vi "IR Opo Main.vi"() -> ()   [LabVIEW 2016]
uses:
  <vilib>/vision/NI_Vision_Development_Module.lvlib
  D:/Fabrizio/Labview Projects/VersionControlled/Laser Ablation Capture Software/uc480DotNet.dll
  Laser Ablation Capture Software/uc480DotNet.dll
  System.Windows.Forms
  <vilib>/Utility/miscctls.llb/LVBoundsTypeDef.ctl
  <vilib>/Utility/config.llb/NI_LVConfig.lvlib
  <vilib>/regexp/Match Regular Expression.xnode
panel:
  in  "Load ROI":bool
  in  "Save current ROI":bool
  in  "Call Last ROI":bool
  in  "Circle?":bool=TRUE
  out "Axis 2 group":i32
  out "Axis 1 group":i32
  in  "Microscope/Capture \nstatus button":bool=TRUE
  in  "X travel":dbl min=0.0 max=50.0 step=0.0001
  in  "Y travel":dbl min=0.0 max=150.0 step=0.0001
  in  "Laser Status":bool
  in  "SINGLE SHOT":bool
  in  "Repetition\nRate (Hz)":dbl=2.34 min=1.0 max=20.0 step=0.01 format="%.2g"
  out "Laser Com Delay":i32
  out "VISA Laser port":string
  in  "Acceleration \n(mm/s²)":dbl=20.0
  out "Camera Status":string="Load parameter"
  in  "Save configuration":bool
  in  "Stages status":bool
  in  "Transparency":u8 max=80 step=1
  in  "Overlay MSI Image":bool
  in  "Home Axes":bool
  out "Axis 2 Offset":dbl
  out "Axis 1 Offset":dbl
  out "Acceleration":dbl
  out "Velocity":dbl
  in  "Axis Initial Parameters":T1={"Velocity (units/seconds)"=1.0, "Acceleration (units/seconds²)"=20.0, "Minimum Jerk Time (seconds)"=0.005, "Maximum Jerk Time (seconds)"=0.009} {"Maximum Jerk Time (seconds)" format="%.6e"; "Minimum Jerk Time (seconds)" format="%.6e"; "Acceleration (units/seconds²)" format="%.6e"; "Velocity (units/seconds)" format="%.6e"}
  out "Axis 2":string
  out "Axis 1":string
  out "XPS_Address":string
  in  "Axes Manual Control":bool
  out "ROI Area \n(mm2)":dbl=4.035870075999999
  out "Laser on/off array":bool[][](array[boolean])
  out "Commands array":string[][](array[string])
  in  "Exit Camera":bool
  in  "Width (px)":i32=240
  in  "Y offset":i32=406 step=1
  in  "X offset":i32=693 step=1
  out "Processi time (sec)":i32=117
  in  "Processing time unit":string(combo)="sec"
  out "Process time":dbl=117.0
  in  "Mode":i32(ring) items=["RGB 32"=0, "RGB 24"=1, "Y8 Monochrom"=6]
  in  "Camera":refnum<k24>(container)
  in  "Init Camera":bool
  in  "Start Live":bool
  in  "Stop Live":bool
  in  "Load Parameter":bool
  out "Error Out":errorcluster caption="error"
  out "Bits/Pixel":i32=32
  out "Width":i32=1280
  out "Height":i32=1024
  out "Serial Number":string="4102944807"
  in  "Camera ID":i32
  in  "Zoom":dbl(ring)=1.5 items=["4X"=4.0, "2X"=2.0, "1.5X"=1.5, "1.25X"=1.25, "1X"=1.0]
  in  "Gain Boost":bool=TRUE
  in  "Snapshot":bool
  out "Output":picture
  in  "Exposure":dbl(slide)=99.80425000000001 min=0.06241666666666667 max=99.80425000000001 step=0.06241666666666667 scale=0.06241666666666667..99.80425000000001 scale format="%#.3g"
  in  "Framerate":dbl(slide)=10.002522802986672 min=0.47411700449083627 max=15.001275108384213 step=0.014032998230481021 scale=0.47411700449083627..15.001275108384213 scale format="%#.3g"
  in  "Pixelclock":i32(slide)=24 min=5 max=40 step=1 scale=5.0..40.0
  in  "error in (no error)":errorcluster
  out "error out":errorcluster
  in  "Precision (%)":dbl=1.0 min=1.0 max=100.0 step=1.0 format="%#_3g"
  in  "Process Image":bool
  in  "Pixel size":dbl=12.19 step=0.01
  in  "Speed (µm/s)":i32=1000
  in  "Heigth (px)":i32=240
  in  "Height  step \ndivider":i32=2
  out "ROI container\nheigth (µm)":i32=2267
  out "ROI container\nwidth (µm)":i32=2267
  out "Source":T2(plugin-control)
  in  "Open \nManual":bool
  in  "Capture":bool
  out "Log":string
  out "Laser Operation":bool
  in  "LASER":bool
  in  "LAMP":bool
  in  "EXIT":bool
  # "Laser Control"
  # "Stages Control"
  # "Camera Control"
  # "ROI Processing"
  # "Laser spot size and position"
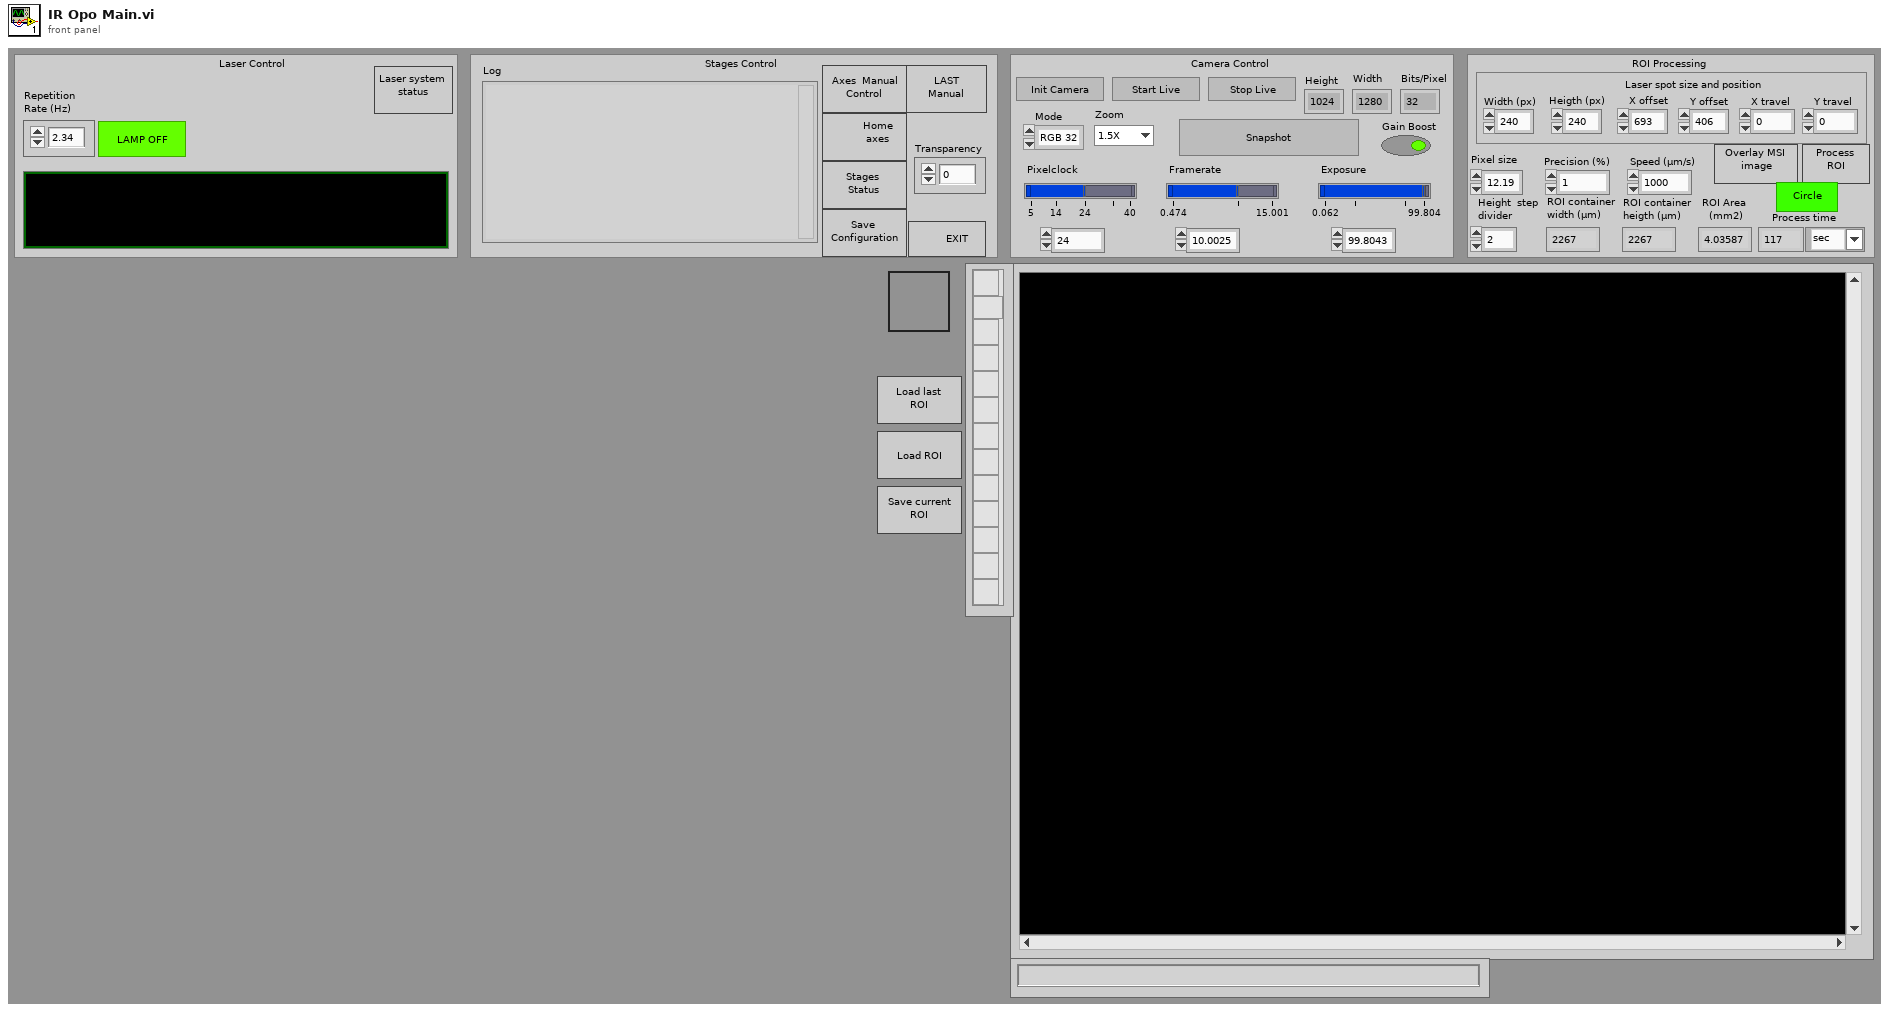
[diagram p1: front panel]
types:
  T1 = cluster{"Velocity (units/seconds)":dbl, "Acceleration (units/seconds²)":dbl, "Minimum Jerk Time (seconds)":dbl, "Maximum Jerk Time (seconds)":dbl}
  T2 = typedef "IMAQ Image.ctl" = refnum<image>
  T3 = typedef "LVBoundsTypeDef.ctl" = cluster{"Width":u32, "Height":u32}
  T4 = enum8{"Enabled", "Disabled", "Disabled and Grayed Out"}
  T5 = typedef "NI_LVConfig.lvlib/Config Data RefNum.ctl" = refnum<k1>
  T6 = enum16{"open", "replace", "create", "open or create", "replace or create", "replace or create with confirmation"}
  T7 = enum32{"Invalid", "Standard", "Closed", "Hidden", "Minimized", "Maximized"}
  T8 = enum32{"invalid app kind", "Development System", "Run Time System", "Student Edition", "Embedded LabVIEW", "Evaluation", "Custom"}
  T9 = cluster{"connection TCP":refnum<k5>, "LogTo File":bool, "Log File refnum":refnum<file>, "no error if error log":bool}
  T10 = typedef "Image Type" = u32
  T11 = cluster{"Global Rectangle":i32[], "Contours":cluster{"Contour Type":u32, "ROI Type":u32, "Points":i32[]}[]}
  T12 = cluster{"Global Rectangle[0]":i32, "Global Rectangle[1]":i32}
  T13 = typedef "ROI Descriptor" = cluster{"Global Rectangle":i32[], "Contours":cluster{"ID":enum32{"External", "Internal"}, "Type":u32, "Coordinates":i32[]}[]}
  T14 = cluster{"ID":enum32{"External", "Internal"}, "Type":u32, "Coordinates":i32[]}[]
  T15 = cluster{"ID":enum32{"External", "Internal"}, "Type":u32, "Coordinates":i32[]}
  T16 = cluster{"Contour Type":u32, "ROI Type":u32, "Points":i32[]}[]
  T17 = cluster{"Contour Type":u32, "ROI Type":u32, "Points":i32[]}
diagram:
  w35 = 1 items=["None", "FixedSingle", "Fixed3D"] ("BorderStyle")
  # "Button and controls"
  # "Camera control buttons"
  n1 = property class="PictureBox"(reference="Camera", "BorderStyle"=w35, "Width"=853, "Height"=682) -> (reference out=w23:refnum<k24>, error out=w24:errorcluster)  [unwired: 1 in]
  n2 = property class="PictureBox"(reference=w23, error in=w24) -> (reference out=w22:refnum<k24>, error out=w21:errorcluster, "Handle"=w20:refnum<k24>)
  n3 = while "Camera Control" {
    shift-right: [w52] -> _
    shift-left: w21 -> [w58]
    shift-right: [w55] -> _
    shift-left: _ -> [w48]
    shift-right: [w50] -> _
    shift-left: w22 -> [w51]
    tunnel: w20 -> [w49]
    stop <- w56 stop-if-true
    # ".NetReference"
    # ".Net Reference"
    n4 = event shown="[1] Timeout" {
      selector: _ -> [_ _]
      dyn-events: _ -> [_ _]
      timeout: 0 -> [_ _]
      event "Load Parameter", "Start Live": Mouse Down {
        n5 = event-data() -> ()  [unwired: 1 in, 2 out]
      }
      event Timeout {
        n6 = event-data() -> ()  [unwired: 1 in, 2 out]
      }
    }
    n7 = event shown="[1] Timeout" {
      selector: _ -> [_ _]
      dyn-events: _ -> [_ _]
      timeout: 0 -> [_ _]
      tunnel: [w72 w83] -> w59
      tunnel: w58 -> [w82 w83]
      tunnel: w48 -> [w81 _]
      event "Pixelclock": Value Change; "Pixelclock": Mouse Move; "Pixelclock": Key Down; "Pixelclock": Mouse Up {
        n8 = event-data() -> ("CtlRef"=w74:refnum<vi>)  [unwired: 1 in, 3 out]
        n9 = call "uc480_SubVI_Example_GetFramerate.vi"(".NET (Reference)"=w81, "Error In"=w82) -> ("Framerate"=w80:dbl, "Inc"=w79:dbl, "Min"=w77:dbl, "Max"=w78:dbl, "error out"=w76:errorcluster)  [unwired: 9 in]
        n10 = property on="Framerate" class="Slide (strict)"(error in=w76, "Value"=w80, "Increment"=w79, "Minimum"=w77, "Maximum"=w78) -> (error out=w75:errorcluster)  [unwired: 1 in, 1 out]
        n11 = property on="Framerate" class="Slide (strict)"(error in=w75, "Scale.Increment"=w79, "Scale.Minimum"=w77, "Scale.Maximum"=w78) -> (error out=w73:errorcluster)  [unwired: 1 in, 1 out]
        n12 = Close Reference(reference=w74, error in (no error)=w73) -> (error out=w72:errorcluster)
      }
      event Timeout {
        n13 = event-data() -> ()  [unwired: 1 in, 2 out]
      }
    }
    n14 = case shown="False" "Load Parameter" {
      tunnel: ["" "Load parameter"] -> w65
      frame False {
      }
      frame True {
      }
    }
    n15 = case shown="False" "Init Camera" {
      tunnel: ["" "Init camera"] -> w69
      frame False {
      }
      frame True {
      }
    }
    n16 = case shown="False" "Exit Camera" {
      tunnel: ["" "Exit camera"] -> w63
      frame False {
      }
      frame True {
      }
    }
    n17 = event shown="[1] Timeout" {
      selector: _ -> [_ _]
      dyn-events: _ -> [_ _]
      timeout: 0 -> [_ _]
      tunnel: w59 -> [w94 w95]
      tunnel: [w84 w95] -> w61
      tunnel: w48 -> [w93 _]
      event "Pixelclock", "Framerate": Value Change; "Pixelclock", "Framerate": Mouse Move; "Pixelclock", "Framerate": Key Down; "Pixelclock", "Framerate": Mouse Up {
        n18 = event-data() -> ("CtlRef"=w86:refnum<vi>)  [unwired: 1 in, 3 out]
        n19 = call "uc480_SubVI_Example_GetExposure.vi"(".NET (Reference)"=w93, "Error In"=w94) -> ("Exposure"=w90:dbl, "Inc"=w89:dbl, "Min"=w88:dbl, "Max"=w87:dbl, "Error out"=w91:errorcluster)  [unwired: 9 in]
        n20 = property on="Exposure" class="Slide (strict)"(error in=w91, "Value"=w90, "Increment"=w89, "Minimum"=w88, "Maximum"=w87) -> (error out=w92:errorcluster)  [unwired: 1 in, 1 out]
        n21 = property on="Exposure" class="Slide (strict)"(error in=w92, "Scale.Increment"=w89, "Scale.Minimum"=w88, "Scale.Maximum"=w87) -> (error out=w85:errorcluster)  [unwired: 1 in, 1 out]
        n22 = Close Reference(reference=w86, error in (no error)=w85) -> (error out=w84:errorcluster)
      }
      event Timeout {
        n23 = event-data() -> ()  [unwired: 1 in, 2 out]
      }
    }
    n24 = case shown="False" "Start Live" {
      tunnel: ["" "Start live"] -> w68
      frame False {
      }
      frame True {
      }
    }
    n25 = case shown="False" "Stop Live" {
      tunnel: ["" "Stop live"] -> w64
      frame False {
      }
      frame True {
      }
    }
    n26 = local read "Camera Status"() -> (w45:string)
    n27 = Concatenate Strings(w69, w68, w65, w64, w63) -> (→"Camera Status":string)
    n28 = case shown="Default" w45 {
      tunnel: w48 -> [w138 w178 w236 w278 w458 w517]
      tunnel: w61 -> [w141 w179 w237 w288 w457 w518]
      tunnel: [w112 w177 w245 w287 w416 w516] -> w55
      tunnel: [w113 w176 w246 w286 w453 w514] -> w54
      tunnel: [FALSE FALSE TRUE FALSE FALSE FALSE] -> w56
      tunnel: w51 -> [w111 w170 w218 w270 w411 w507]
      tunnel: [w111 w170 w217 w269 w411 w507] -> w50
      tunnel: w49 -> [_ _ _ w266 _ _]
      frame "Load parameter" {
        # "SubVI Example for \nMemory allocation"
        # "Is acquisition running?"
        # "Load Parameter"
        n29 = property class="Camera"(reference=w138, error in=w141) -> (error out=w146:errorcluster, "Acquisition"=w145:refnum<k24>)  [unwired: 1 out]
        n30 = invoke class="Acquisition" method="HasStarted"(reference=w145, error in=w146) -> (reference out=w142:refnum<k24>, error out=w144:errorcluster, "bValue"=w140:bool)  [unwired: 2 in, 1 out]
        n31 = control-ref of="Start Live"() -> (w136:refnum<vi>)
        n32 = invoke class="Acquisition" method="ToString"(reference=w142, error in=w144) -> (reference out=w108:refnum<k24>, error out=w107:errorcluster, "ToString"=w143:string)  [unwired: 1 in]
        n33 = property class="Bool"(reference=w136, "Disabled"=u8 0 ("Deaktiviert")) -> (reference out=w110:refnum<vi>, error out=w109:errorcluster)  [unwired: 1 in]
        n34 = Close Reference(reference=w108, error in (no error)=w107) -> (error out=w106:errorcluster)
        n35 = Close Reference(reference=w110, error in (no error)=w109) -> ()  [unwired: 1 out]
        n36 = call "uc480_Error_Handling.vi"("Error String"=w143, "Error In"=w106) -> ("Error Out"=w139:errorcluster)  [unwired: 9 in]
        n37 = case shown="False" w140 {
          tunnel: w139 -> [w154 w161]
          tunnel: w138 -> [w152 w162]
          tunnel: [w153 w161] -> w137
          tunnel: [w152 w162] -> w112
          frame False {
            n38 = property class="Camera"(reference=w152, error in=w154) -> (error out=w156:errorcluster, "Parameter"=w155:refnum<k24>)  [unwired: 1 out]
            n39 = invoke class="Parameter" method="Load"(reference=w155, error in=w156, "strFilename"="") -> (reference out=w158:refnum<k24>, error out=w159:errorcluster, "Load"=w151:i32)  [unwired: 1 in, 1 out]
            n40 = invoke class="Parameter" method="ToString"(reference=w158, error in=w159) -> (reference out=w148:refnum<k24>, error out=w150:errorcluster, "ToString"=w160:string)  [unwired: 1 in]
            n41 = Close Reference(reference=w148, error in (no error)=w150) -> (error out=w149:errorcluster)
            n42 = call "uc480_Error_Handling.vi"("Error Code"=w151, "Error String"=w160, "Error In"=w149) -> ("Error Out"=w153:errorcluster)  [unwired: 8 in]
          }
          frame True {
          }
        }
        n43 = call "uc480_SubVI_Example_MemoryAllocation.vi"(".NET (Reference)"=w112, "Error In"=w137) -> ("Error Out"=w114:errorcluster)  [unwired: 13 in, 4 out]
        n44 = call "uc480_SubVI_Example_GetPixelClock.vi"(".NET (Reference)"=w112, "Error In"=w114) -> ("Pixel Clock"=w115:i32, "Inc"=w117:i32, "Min"=w118:i32, "Max"=w119:i32, "error out"=w116:errorcluster)  [unwired: 9 in]
        n45 = property on="Pixelclock" class="Slide (strict)"(error in=w116, "Value"=w115, "Increment"=w117, "Minimum"=w118, "Maximum"=w119) -> (error out=w120:errorcluster)  [unwired: 1 in, 1 out]
        n46 = property on="Pixelclock" class="Slide (strict)"(error in=w120, "Scale.Increment"=w117, "Scale.Minimum"=w118, "Scale.Maximum"=w119) -> (error out=w121:errorcluster)  [unwired: 1 in, 1 out]
        n47 = call "uc480_SubVI_Example_GetFramerate.vi"(".NET (Reference)"=w112, "Error In"=w121) -> ("Framerate"=w124:dbl, "Inc"=w125:dbl, "Min"=w126:dbl, "Max"=w127:dbl, "error out"=w123:errorcluster)  [unwired: 9 in]
        n48 = property on="Framerate" class="Slide (strict)"(error in=w123, "Value"=w124, "Increment"=w125, "Minimum"=w126, "Maximum"=w127) -> (error out=w122:errorcluster)  [unwired: 1 in, 1 out]
        n49 = property on="Framerate" class="Slide (strict)"(error in=w122, "Scale.Increment"=w125, "Scale.Minimum"=w126, "Scale.Maximum"=w127) -> (error out=w128:errorcluster)  [unwired: 1 in, 1 out]
        n50 = call "uc480_SubVI_Example_GetExposure.vi"(".NET (Reference)"=w112, "Error In"=w128) -> ("Exposure"=w131:dbl, "Inc"=w132:dbl, "Min"=w133:dbl, "Max"=w134:dbl, "Error out"=w129:errorcluster)  [unwired: 9 in]
        n51 = property on="Exposure" class="Slide (strict)"(error in=w129, "Value"=w131, "Increment"=w132, "Minimum"=w133, "Maximum"=w134) -> (error out=w130:errorcluster)  [unwired: 1 in, 1 out]
        n52 = property on="Exposure" class="Slide (strict)"(error in=w130, "Scale.Increment"=w132, "Scale.Minimum"=w133, "Scale.Maximum"=w134) -> (error out=w113:errorcluster)  [unwired: 1 in, 1 out]
      }
      frame "Stop live" {
        # "Is acquisition running?"
        # "Stop Acquisition"
        n53 = property class="Camera"(reference=w178, error in=w179) -> (error out=w186:errorcluster, "Acquisition"=w185:refnum<k24>)  [unwired: 1 out]
        n54 = invoke class="Acquisition" method="HasStarted"(reference=w185, error in=w186) -> (reference out=w180:refnum<k24>, error out=w182:errorcluster, "bValue"=w184:bool)  [unwired: 2 in, 1 out]
        n55 = control-ref of="Load Parameter"() -> (w174:refnum<vi>)
        n56 = control-ref of="Start Live"() -> (w171:refnum<vi>)
        n57 = invoke class="Acquisition" method="ToString"(reference=w180, error in=w182) -> (reference out=w163:refnum<k24>, error out=w165:errorcluster, "ToString"=w181:string)  [unwired: 1 in]
        n58 = property class="Bool"(reference=w174, "Disabled"=u8 0 ("Deaktiviert")) -> (reference out=w169:refnum<vi>, error out=w168:errorcluster)  [unwired: 1 in]
        n59 = property class="Bool"(reference=w171, "Disabled"=u8 0 ("Deaktiviert")) -> (reference out=w167:refnum<vi>, error out=w166:errorcluster)  [unwired: 1 in]
        n60 = Close Reference(reference=w163, error in (no error)=w165) -> (error out=w164:errorcluster)
        n61 = Close Reference(reference=w169, error in (no error)=w168) -> ()  [unwired: 1 out]
        n62 = Close Reference(reference=w167, error in (no error)=w166) -> ()  [unwired: 1 out]
        n63 = call "uc480_Error_Handling.vi"("Error String"=w181, "Error In"=w164) -> ("Error Out"=w183:errorcluster)  [unwired: 9 in]
        n64 = case shown="True" w184 {
          tunnel: [w188 w207] -> w176
          tunnel: w183 -> [w188 w208]
          tunnel: w178 -> [w187 w200]
          tunnel: [w187 w200] -> w177
          frame False {
          }
          frame True {
            n65 = property class="Camera"(reference=w200, error in=w208) -> (error out=w204:errorcluster, "Acquisition"=w205:refnum<k24>)  [unwired: 1 out]
            n66 = invoke class="Acquisition" method="Stop"(reference=w205, error in=w204) -> (reference out=w202:refnum<k24>, error out=w203:errorcluster, "Stop"=w201:i32)  [unwired: 1 in]
            n67 = invoke class="Acquisition" method="ToString"(reference=w202, error in=w203) -> (reference out=w197:refnum<k24>, error out=w199:errorcluster, "ToString"=w206:string)  [unwired: 1 in]
            n68 = Close Reference(reference=w197, error in (no error)=w199) -> (error out=w198:errorcluster)
            n69 = call "uc480_Error_Handling.vi"("Error Code"=w201, "Error String"=w206, "Error In"=w198) -> ("Error Out"=w207:errorcluster)  [unwired: 8 in]
            n70 = Get Date/Time In Seconds() -> (seconds since 1Jan1904=w195:timestamp)
            n71 = Format Date/Time String(time format string (%c)="%m/%d/%y - %I:%M %p  ", seconds (now)=w195) -> (date/time string=w196:string)  [unwired: 1 in]
            n72 = Concatenate Strings(w196, "Camera stopped", "\r") -> (w191:string)
            n73 = invoke on="Log" class="Str" method="Append String"("string"=w191) -> (error out=w189:errorcluster)  [unwired: 3 in, 3 out]
            n74 = property on="Log" class="Str"(error in=w189, "Text.Scroll Position"=u32 500000) -> ()  [unwired: 1 in, 2 out]
          }
        }
      }
      frame "Exit camera" {
        # "Close .Net Reference"
        # "Is acquisition running?"
        # "Stop Acquisition"
        # "Close Camera"
        n75 = property class="Camera"(reference=w236, error in=w237) -> (error out=w244:errorcluster, "Acquisition"=w243:refnum<k24>)  [unwired: 1 out]
        n76 = invoke class="Acquisition" method="HasStarted"(reference=w243, error in=w244) -> (reference out=w238:refnum<k24>, error out=w240:errorcluster, "bValue"=w242:bool)  [unwired: 2 in, 1 out]
        n77 = control-ref of="Load Parameter"() -> (w227:refnum<vi>)
        n78 = control-ref of="Init Camera"() -> (w229:refnum<vi>)
        n79 = control-ref of="Start Live"() -> (w228:refnum<vi>)
        n80 = control-ref of="Stop Live"() -> (w226:refnum<vi>)
        n81 = invoke class="Acquisition" method="ToString"(reference=w238, error in=w240) -> (reference out=w223:refnum<k24>, error out=w225:errorcluster, "ToString"=w239:string)  [unwired: 1 in]
        n82 = property class="Bool"(reference=w228, "Disabled"=u8 0 ("Deaktiviert")) -> (reference out=w212:refnum<vi>, error out=w211:errorcluster)  [unwired: 1 in]
        n83 = property class="Bool"(reference=w229, "Disabled"=u8 0 ("Deaktiviert")) -> (reference out=w210:refnum<vi>, error out=w209:errorcluster)  [unwired: 1 in]
        n84 = property class="Bool"(reference=w227, "Disabled"=u8 0 ("Deaktiviert")) -> (reference out=w214:refnum<vi>, error out=w213:errorcluster)  [unwired: 1 in]
        n85 = property class="Bool"(reference=w226, "Disabled"=u8 0 ("Deaktiviert")) -> (reference out=w216:refnum<vi>, error out=w215:errorcluster)  [unwired: 1 in]
        n86 = Close Reference ("Close Referenz")(reference=w223, error in (no error)=w225) -> (error out=w224:errorcluster)
        n87 = Close Reference(reference=w212, error in (no error)=w211) -> ()  [unwired: 1 out]
        n88 = Close Reference(reference=w210, error in (no error)=w209) -> ()  [unwired: 1 out]
        n89 = Close Reference(reference=w216, error in (no error)=w215) -> ()  [unwired: 1 out]
        n90 = Close Reference(reference=w214, error in (no error)=w213) -> ()  [unwired: 1 out]
        n91 = call "uc480_Error_Handling.vi"("Error String"=w239, "Error In"=w224) -> ("Error Out"=w241:errorcluster)  [unwired: 9 in]
        n92 = case shown="True" w242 {
          tunnel: [w253 w264] -> w234
          tunnel: w241 -> [w253 w265]
          tunnel: w236 -> [w252 w257]
          tunnel: [w252 w257] -> w235
          frame False {
          }
          frame True {
            n93 = property class="Camera"(reference=w257, error in=w265) -> (error out=w261:errorcluster, "Acquisition"=w262:refnum<k24>)  [unwired: 1 out]
            n94 = invoke class="Acquisition" method="Stop"(reference=w262, error in=w261) -> (reference out=w259:refnum<k24>, error out=w260:errorcluster, "Stop"=w258:i32)  [unwired: 1 in]
            n95 = invoke class="Acquisition" method="ToString"(reference=w259, error in=w260) -> (reference out=w254:refnum<k24>, error out=w256:errorcluster, "ToString"=w263:string)  [unwired: 1 in]
            n96 = Close Reference ("Close Referenz")(reference=w254, error in (no error)=w256) -> (error out=w255:errorcluster)
            n97 = call "uc480_Error_Handling.vi"("Error Code"=w258, "Error String"=w263, "Error In"=w255) -> ("Error Out"=w264:errorcluster)  [unwired: 8 in]
          }
        }
        n98 = invoke class="Camera" method="Exit"(reference=w235, error in=w234) -> (reference out=w245:refnum<k24>, error out=w248:errorcluster, "Exit"=w247:i32)  [unwired: 1 in]
        n99 = invoke class="Camera" method="ToString"(reference=w245, error in=w248) -> (error out=w249:errorcluster, "ToString"=w250:string)  [unwired: 1 in, 1 out]
        n100 = call "uc480_Error_Handling.vi"("Error Code"=w247, "Error String"=w250, "Error In"=w249) -> ("Error Out"=w222:errorcluster)  [unwired: 8 in]
        n101 = property class="PictureBox"(reference=w218, error in=w222, "Width"=853, "Height"=682) -> (reference out=w217:refnum<k24>, error out=w221:errorcluster)
        n102 = Close Reference ("Close Referenz")(reference=w245, error in (no error)=w221) -> (error out=w246:errorcluster)
      }
      frame Default {
        # "SubVI Example for Timing"
        # "Has acquisition started?"
        n103 = call "uc480_SubVI_Example_Timing.vi"(".NET (Reference)"=w278, "Pixelclock"="Pixelclock", "Exposure time"="Exposure", "Framerate"="Framerate", "Error In"=w288) -> ("Pixelclock"=w281:i32, "Exposure time"=w280:dbl, "Framerate"=w279:dbl, "Error Out"=w285:errorcluster)  [unwired: 7 in]
        n104 = property on="Framerate" class="Schieber (strikt)"(error in=w285, "Scale.RngStart"=w279) -> (error out=w284:errorcluster)  [unwired: 1 in, 1 out]
        n105 = property on="Exposure" class="Schieber (strikt)"(error in=w284, "Scale.RngStart"=w280) -> (error out=w283:errorcluster)  [unwired: 1 in, 1 out]
        n106 = property on="Pixelclock" class="Schieber (strikt)"(error in=w283, "Scale.RngStart"=w281) -> (error out=w282:errorcluster)  [unwired: 1 in, 1 out]
        n107 = property class="Camera"(reference=w278, error in=w282) -> (reference out=w271:refnum<k24>, error out=w294:errorcluster, "Acquisition"=w293:refnum<k24>)
        n108 = invoke class="Acquisition" method="HasStarted"(reference=w293, error in=w294) -> (reference out=w268:refnum<k24>, error out=w290:errorcluster, "HasStarted"=w289:i32, "bValue"=w267:bool)  [unwired: 2 in]
        n109 = invoke class="Acquisition" method="ToString"(reference=w268, error in=w290) -> (reference out=w272:refnum<k24>, error out=w292:errorcluster, "ToString"=w291:string)  [unwired: 1 in]
        n110 = call "uc480_Error_Handling.vi"("Error Code"=w289, "Error String"=w291, "Error In"=w292) -> ("Error Out"=w274:errorcluster)  [unwired: 8 in]
        n111 = Close Reference(reference=w272, error in (no error)=w274) -> (error out=w273:errorcluster)
        n112 = case "Show Image" shown="True" w267 {
          tunnel: [w298 w310] -> w286
          tunnel: w273 -> [w298 w338]
          tunnel: w271 -> [w297 w302]
          tunnel: [w297 w306] -> w287
          tunnel: w270 -> [w296 w327]
          tunnel: [w296 w304] -> w269
          tunnel: w266 -> [_ w334]
          frame False {
            (unwired) ""
          }
          frame True {
            n113 = local read "Height"() -> (w331:i32)
            n114 = local read "Width"() -> (w332:i32)
            n115 = Quotient & Remainder(x=w332, y="Zoom") -> (floor(x/y)=w329:dbl)  [unwired: 1 out]
            n116 = Quotient & Remainder(x=w331, y="Zoom") -> (floor(x/y)=w328:dbl)  [unwired: 1 out]
            n117 = To Long Integer(number=w329) -> (32bit integer=w301:i32)
            n118 = To Long Integer(number=w328) -> (32bit integer=w300:i32)
            n119 = property class="PictureBox"(reference=w327, error in=w338, "Width"=w301, "Height"=w300) -> (reference out=w304:refnum<k24>, error out=w333:errorcluster)
            n120 = property class="Camera"(reference=w302, error in=w333) -> (reference out=w303:refnum<k24>, error out=w340:errorcluster, "Memory"=w341:refnum<k24>)
            n121 = invoke class="Memory" method="GetActive"(reference=w341, error in=w340) -> (reference out=w335:refnum<k24>, error out=w336:errorcluster, "s32MemId"=w307:i32)  [unwired: 2 in, 1 out]
            n122 = property class="Camera"(reference=w303, error in=w336) -> (reference out=w315:refnum<k24>, error out=w339:errorcluster, "Display"=w324:refnum<k24>)
            n123 = invoke class="Display" method="Render"(reference=w324, error in=w339, "memID"=w307, "windowHandle"=w334) -> (reference out=w325:refnum<k24>, error out=w326:errorcluster)  [unwired: 1 in, 3 out]
            n124 = property class="Camera"(reference=w315, error in=w326) -> (reference out=w306:refnum<k24>, error out=w322:errorcluster, "Gain"=w320:refnum<k24>)
            n125 = property class="Gain"(reference=w320, error in=w322) -> (reference out=w321:refnum<k24>, error out=w317:errorcluster, "Hardware"=w316:refnum<k24>)
            n126 = property class="GainHardware"(reference=w316, error in=w317) -> (reference out=w313:refnum<k24>, error out=w318:errorcluster, "Boost"=w319:refnum<k24>)
            n127 = property class="GainBoost"(reference=w319, error in=w318, "Enabled"="Gain Boost") -> (reference out=w314:refnum<k24>, error out=w305:errorcluster)
            n128 = case "Snapshot control" shown="True" "Snapshot" {
              tunnel: w302 -> [_ w362]
              tunnel: w305 -> [w342 w366]
              tunnel: [w342 w353] -> w299
              tunnel: w301 -> [_ w356]
              tunnel: w300 -> [_ w355]
              frame False {
              }
              frame True {
                n129 = property class="Camera"(reference=w362, error in=w366) -> (error out=w386:errorcluster, "Memory"=w385:refnum<k24>)  [unwired: 1 out]
                n130 = local read "Zoom"() -> (w361:dbl)
                n131 = invoke class="Memory" method="GetList"(reference=w385, error in=w386) -> (reference out=w391:refnum<k24>, error out=w390:errorcluster, "GetList"=w392:i32, "idList"=w379:i32[])  [unwired: 2 in]
                n132 = Bundle(cluster=T3 {"Width"=0, "Height"=0} ("Draw Area Size"), "Width"=w356, "Height"=w355) -> (w357:T3)
                n133 = Divide(x=1.0, y=w361) -> (x/y=w359:dbl)
                n134 = property on="Output" class="Pict"("ZoomFactor"=w359, "Draw Area Size"=w357) -> ()  [unwired: 2 in, 2 out]
                n135 = invoke class="Memory" method="ToString"(reference=w391, error in=w390) -> (reference out=w364:refnum<k24>, error out=w374:errorcluster, "ToString"=w389:string)  [unwired: 1 in]
                n136 = Index Array(array=w379, index=0 ("Active \nAcquisition Buffer")) -> (element=w376:i32)
                n137 = Index Array(array=w379, index=u32 0 ("Active \nOutput Buffer")) -> (element=w375:i32)
                n138 = Close Reference(reference=w364, error in (no error)=w374) -> (error out=w373:errorcluster)
                n139 = call "uc480_Error_Handling.vi"("Error Code"=w392, "Error String"=w389, "Error In"=w373) -> ("Error Out"=w382:errorcluster)  [unwired: 8 in]
                n140 = Get Date/Time In Seconds() -> (seconds since 1Jan1904=w346:timestamp)
                n141 = property class="Camera"(reference=w362, error in=w382) -> (error out=w381:errorcluster, "Memory"=w380:refnum<k24>)  [unwired: 1 out]
                n142 = Format Date/Time String(time format string (%c)="%m/%d/%y -%I:%M %p  ", seconds (now)=w346) -> (date/time string=w345:string)  [unwired: 1 in]
                n143 = invoke class="Memory" method="SetActive"(reference=w380, error in=w381, "s32MemId"=w376) -> (reference out=w365:refnum<k24>, error out=w372:errorcluster)  [unwired: 1 in, 2 out]
                n144 = Concatenate Strings(w345, "Snapshot taken", "\r") -> (w350:string)
                n145 = Close Reference(reference=w365, error in (no error)=w372) -> (error out=w371:errorcluster)
                n146 = invoke on="Log" class="Str" method="Append String"("string"=w350) -> (error out=w343:errorcluster)  [unwired: 3 in, 3 out]
                n147 = property class="Camera"(reference=w362, error in=w371) -> (error out=w388:errorcluster, "Memory"=w377:refnum<k24>)  [unwired: 1 out]
                n148 = invoke class="Memory" method="CopyToArray"(reference=w377, error in=w388, "s32MemId"=w375) -> (reference out=w367:refnum<k24>, error out=w368:errorcluster, "u8Image"=w387:u8[])  [unwired: 2 in, 2 out]
                n149 = property on="Log" class="Str"(error in=w343, "Text.Scroll Position"=u32 500000) -> ()  [unwired: 1 in, 2 out]
                n150 = invoke class="Memory" method="ToString"(reference=w367, error in=w368) -> (reference out=w363:refnum<k24>, error out=w370:errorcluster, "ToString"=w393:string)  [unwired: 1 in]
                n151 = Close Reference(reference=w363, error in (no error)=w370) -> (error out=w369:errorcluster)
                n152 = call "uc480_Error_Handling.vi"("Error String"=w393, "Error In"=w369) -> ("Error Out"=w384:errorcluster)  [unwired: 9 in]
                n153 = call "uc480_ArrayToImage.vi"("Error In"=w384, "InArray"=w387, ".NET (Reference)"=w362) -> ("Error Out"=w352:errorcluster, "Image"=w354:picture)  [unwired: 7 in]
                "Output" <- w354
                n154 = call "Picture to IMAQ.vi"("Error In"=w352, "picture"=w354) -> ("Error Out"=w353:errorcluster, "Image"=→"Source":T2)  [unwired: 8 in]
              }
            }
            n155 = Close Reference(reference=w313, error in (no error)=w299) -> (error out=w312:errorcluster)
            n156 = Close Reference(reference=w314, error in (no error)=w312) -> (error out=w309:errorcluster)
            n157 = Close Reference(reference=w321, error in (no error)=w309) -> (error out=w323:errorcluster)
            n158 = Close Reference(reference=w325, error in (no error)=w323) -> (error out=w337:errorcluster)
            n159 = Close Reference(reference=w335, error in (no error)=w337) -> (error out=w310:errorcluster)
          }
        }
      }
      frame "Init camera" {
        # "SubVI Example for \nGetDefault Timing"
        # "SubVI Example for \nMemory allocation"
        # "SubVI Example for \nTiming"
        # "SubVI Example for \nCamera Init"
        # "Pixelformat"
        n160 = control-ref of="Load Parameter"() -> (w417:refnum<vi>)
        n161 = call "uc480_SubVI_Example_CameraInit.vi"("Error In"=w457, "Camera ID"="Camera ID", "Init Camera Flag"=TRUE, ".NET (Reference)"=w458) -> ("Error Out"=w463:errorcluster, ".NET (Reference)"=w416:refnum<k24>)  [unwired: 6 in]
        n162 = control-ref of="Init Camera"() -> (w421:refnum<vi>)
        n163 = control-ref of="Start Live"() -> (w419:refnum<vi>)
        n164 = property on="Property Node" class="Camera"(reference=w416, error in=w463) -> (error out=w464:errorcluster, "PixelFormat"=w465:refnum<k24>)  [unwired: 1 out]
        n165 = property class="Bool"(reference=w419, "Disabled"=u8 0 ("Deaktiviert")) -> (reference out=w408:refnum<vi>, error out=w407:errorcluster)  [unwired: 1 in]
        n166 = property class="Bool"(reference=w421, "Disabled"=u8 2 ("Deaktiviert")) -> (reference out=w410:refnum<vi>, error out=w409:errorcluster)  [unwired: 1 in]
        n167 = property class="Bool"(reference=w417, "Disabled"=u8 0 ("Deaktiviert")) -> (reference out=w406:refnum<vi>, error out=w405:errorcluster)  [unwired: 1 in]
        n168 = Close Reference(reference=w408, error in (no error)=w407) -> ()  [unwired: 1 out]
        n169 = Close Reference(reference=w410, error in (no error)=w409) -> ()  [unwired: 1 out]
        n170 = Close Reference(reference=w406, error in (no error)=w405) -> ()  [unwired: 1 out]
        n171 = invoke class="PixelFormat" method="Set"(reference=w465, error in=w464, "mode"="Mode") -> (reference out=w461:refnum<k24>, error out=w454:errorcluster, "Set"=w460:i32)  [unwired: 1 in, 1 out]
        n172 = Get Date/Time In Seconds() -> (seconds since 1Jan1904=w397:timestamp)
        n173 = Format Date/Time String(time format string (%c)="%m/%d/%y - %I:%M %p  ", seconds (now)=w397) -> (date/time string=w396:string)  [unwired: 1 in]
        n174 = invoke class="PixelFormat" method="ToString"(reference=w461, error in=w454) -> (reference out=w402:refnum<k24>, error out=w404:errorcluster, "ToString"=w462:string)  [unwired: 1 in]
        n175 = Concatenate Strings(w396, "Camera Initialized", "\r") -> (w401:string)
        n176 = Close Reference(reference=w402, error in (no error)=w404) -> (error out=w403:errorcluster)
        n177 = call "uc480_Error_Handling.vi"("Error Code"=w460, "Error String"=w462, "Error In"=w403) -> ("Error Out"=w428:errorcluster)  [unwired: 8 in]
        n178 = invoke on="Log" class="Str" method="Append String"("string"=w401) -> (error out=w394:errorcluster)  [unwired: 3 in, 3 out]
        n179 = property on="Log" class="Str"(error in=w394, "Text.Scroll Position"=u32 500000) -> ()  [unwired: 1 in, 2 out]
        n180 = call "uc480_SubVI_Example_GetDefault_Timing.vi"(".NET (Reference)"=w416, "Error In"=w428) -> ("Pixelclock"=w427:i32, "Exposure time"=w426:dbl, "Framerate"=w425:dbl, "Error Out"=w424:errorcluster)  [unwired: 10 in]
        n181 = call "uc480_SubVI_Example_GetPixelClock.vi"(".NET (Reference)"=w416, "Error In"=w424) -> ("Pixel Clock"=w429:i32, "Inc"=w431:i32, "Min"=w432:i32, "Max"=w433:i32, "error out"=w430:errorcluster)  [unwired: 9 in]
        n182 = property on="Pixelclock" class="Slide (strict)"(error in=w430, "Value"=w429, "Increment"=w431, "Minimum"=w432, "Maximum"=w433) -> (error out=w434:errorcluster)  [unwired: 1 in, 1 out]
        n183 = property on="Pixelclock" class="Slide (strict)"(error in=w434, "Scale.Increment"=w431, "Scale.Minimum"=w432, "Scale.Maximum"=w433) -> (error out=w435:errorcluster)  [unwired: 1 in, 1 out]
        n184 = call "uc480_SubVI_Example_GetFramerate.vi"(".NET (Reference)"=w416, "Error In"=w435) -> ("Framerate"=w438:dbl, "Inc"=w439:dbl, "Min"=w440:dbl, "Max"=w441:dbl, "error out"=w437:errorcluster)  [unwired: 9 in]
        n185 = property on="Framerate" class="Slide (strict)"(error in=w437, "Value"=w438, "Increment"=w439, "Minimum"=w440, "Maximum"=w441) -> (error out=w436:errorcluster)  [unwired: 1 in, 1 out]
        n186 = property on="Framerate" class="Slide (strict)"(error in=w436, "Scale.Increment"=w439, "Scale.Minimum"=w440, "Scale.Maximum"=w441) -> (error out=w442:errorcluster)  [unwired: 1 in, 1 out]
        n187 = call "uc480_SubVI_Example_GetExposure.vi"(".NET (Reference)"=w416, "Error In"=w442) -> ("Exposure"=w445:dbl, "Inc"=w446:dbl, "Min"=w447:dbl, "Max"=w448:dbl, "Error out"=w443:errorcluster)  [unwired: 9 in]
        n188 = property on="Exposure" class="Slide (strict)"(error in=w443, "Value"=w445, "Increment"=w446, "Minimum"=w447, "Maximum"=w448) -> (error out=w444:errorcluster)  [unwired: 1 in, 1 out]
        n189 = property on="Exposure" class="Slide (strict)"(error in=w444, "Scale.Increment"=w446, "Scale.Minimum"=w447, "Scale.Maximum"=w448) -> (error out=w423:errorcluster)  [unwired: 1 in, 1 out]
        n190 = call "uc480_SubVI_Example_Timing.vi"(".NET (Reference)"=w416, "Pixelclock"=w427, "Exposure time"=w426, "Framerate"=w425, "Error In"=w423) -> ("Error Out"=w415:errorcluster)  [unwired: 7 in, 3 out]
        n191 = call "uc480_SubVI_Example_Is_XS.vi"("Error In"=w415, ".NET (Reference)"=w416) -> ("Error Out"=w412:errorcluster, "IsXS"=w414:bool)  [unwired: 7 in, 1 out]
        n192 = case shown="False" w414 {
          tunnel: w412 -> [w479 w492]
          tunnel: [w479 w492] -> w413
          frame False {
            n193 = control-ref of="Pixelclock"() -> (w475:refnum<vi>)
            n194 = control-ref of="Framerate"() -> (w474:refnum<vi>)
            n195 = control-ref of="Exposure"() -> (w473:refnum<vi>)
            n196 = property class="Slide (strict)"(reference=w475, "DisabledEnum"=T4."Enabled" ("Disabled")) -> (reference out=w472:refnum<vi>, error out=w471:errorcluster)  [unwired: 1 in]
            n197 = property class="Slide (strict)"(reference=w474, "DisabledEnum"=T4."Enabled" ("Disabled")) -> (reference out=w470:refnum<vi>, error out=w469:errorcluster)  [unwired: 1 in]
            n198 = property class="Slide (strict)"(reference=w473, "DisabledEnum"=T4."Enabled" ("Disabled")) -> (reference out=w468:refnum<vi>, error out=w467:errorcluster)  [unwired: 1 in]
            n199 = Close Reference(reference=w472, error in (no error)=w471) -> ()  [unwired: 1 out]
            n200 = Close Reference(reference=w470, error in (no error)=w469) -> ()  [unwired: 1 out]
            n201 = Close Reference(reference=w468, error in (no error)=w467) -> ()  [unwired: 1 out]
          }
          frame True {
            n202 = control-ref of="Pixelclock"() -> (w491:refnum<vi>)
            n203 = control-ref of="Framerate"() -> (w488:refnum<vi>)
            n204 = control-ref of="Exposure"() -> (w486:refnum<vi>)
            n205 = property class="Slide (strict)"(reference=w491, "DisabledEnum"=T4."Disabled and Grayed Out" ("Disabled")) -> (reference out=w484:refnum<vi>, error out=w485:errorcluster)  [unwired: 1 in]
            n206 = property class="Slide (strict)"(reference=w488, "DisabledEnum"=T4."Disabled and Grayed Out" ("Disabled")) -> (reference out=w483:refnum<vi>, error out=w482:errorcluster)  [unwired: 1 in]
            n207 = property class="Slide (strict)"(reference=w486, "DisabledEnum"=T4."Disabled and Grayed Out" ("Disabled")) -> (reference out=w481:refnum<vi>, error out=w480:errorcluster)  [unwired: 1 in]
            n208 = Close Reference(reference=w484, error in (no error)=w485) -> ()  [unwired: 1 out]
            n209 = Close Reference(reference=w483, error in (no error)=w482) -> ()  [unwired: 1 out]
            n210 = Close Reference(reference=w481, error in (no error)=w480) -> ()  [unwired: 1 out]
          }
        }
        n211 = call "uc480_SubVI_Example_MemoryAllocation.vi"(".NET (Reference)"=w416, "Error In"=w413) -> ("Bits/Pixel 2"=→"Bits/Pixel":i32, "Width"=→"Width":i32, "Serial Number"=→"Serial Number":string, "Height"=→"Height":i32, "Error Out"=w453:errorcluster)  [unwired: 13 in]
      }
      frame "Start live" {
        # "Has acquisition started?"
        # "Start Acquisition"
        n212 = property class="Camera"(reference=w517, error in=w518) -> (error out=w527:errorcluster, "Acquisition"=w526:refnum<k24>)  [unwired: 1 out]
        n213 = invoke class="Acquisition" method="HasStarted"(reference=w526, error in=w527) -> (reference out=w522:refnum<k24>, error out=w521:errorcluster, "HasStarted"=w520:i32, "bValue"=w525:bool)  [unwired: 2 in]
        n214 = control-ref of="Load Parameter"() -> (w510:refnum<vi>)
        n215 = control-ref of="Stop Live"() -> (w508:refnum<vi>)
        n216 = control-ref of="Start Live"() -> (w513:refnum<vi>)
        n217 = property class="Bool"(reference=w513, "Disabled"=u8 2 ("Deaktiviert")) -> (reference out=w502:refnum<vi>, error out=w501:errorcluster)  [unwired: 1 in]
        n218 = property class="Bool"(reference=w510, "Disabled"=u8 2 ("Deaktiviert")) -> (reference out=w504:refnum<vi>, error out=w503:errorcluster)  [unwired: 1 in]
        n219 = invoke class="Acquisition" method="ToString"(reference=w522, error in=w521) -> (error out=w524:errorcluster, "ToString"=w523:string)  [unwired: 1 in, 1 out]
        n220 = property class="Bool"(reference=w508, "Disabled"=u8 0 ("Deaktiviert")) -> (reference out=w506:refnum<vi>, error out=w505:errorcluster)  [unwired: 1 in]
        n221 = call "uc480_Error_Handling.vi"("Error Code"=w520, "Error String"=w523, "Error In"=w524) -> ("Error Out"=w519:errorcluster)  [unwired: 8 in]
        n222 = Close Reference(reference=w506, error in (no error)=w505) -> ()  [unwired: 1 out]
        n223 = Close Reference(reference=w502, error in (no error)=w501) -> ()  [unwired: 1 out]